vi "TLB Native Dynamic Events ver 0.26bvi.vi"() -> ()   [LabVIEW 2018] (continued)
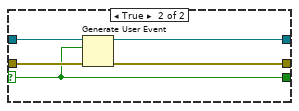
[diagram p2: hidden frame]
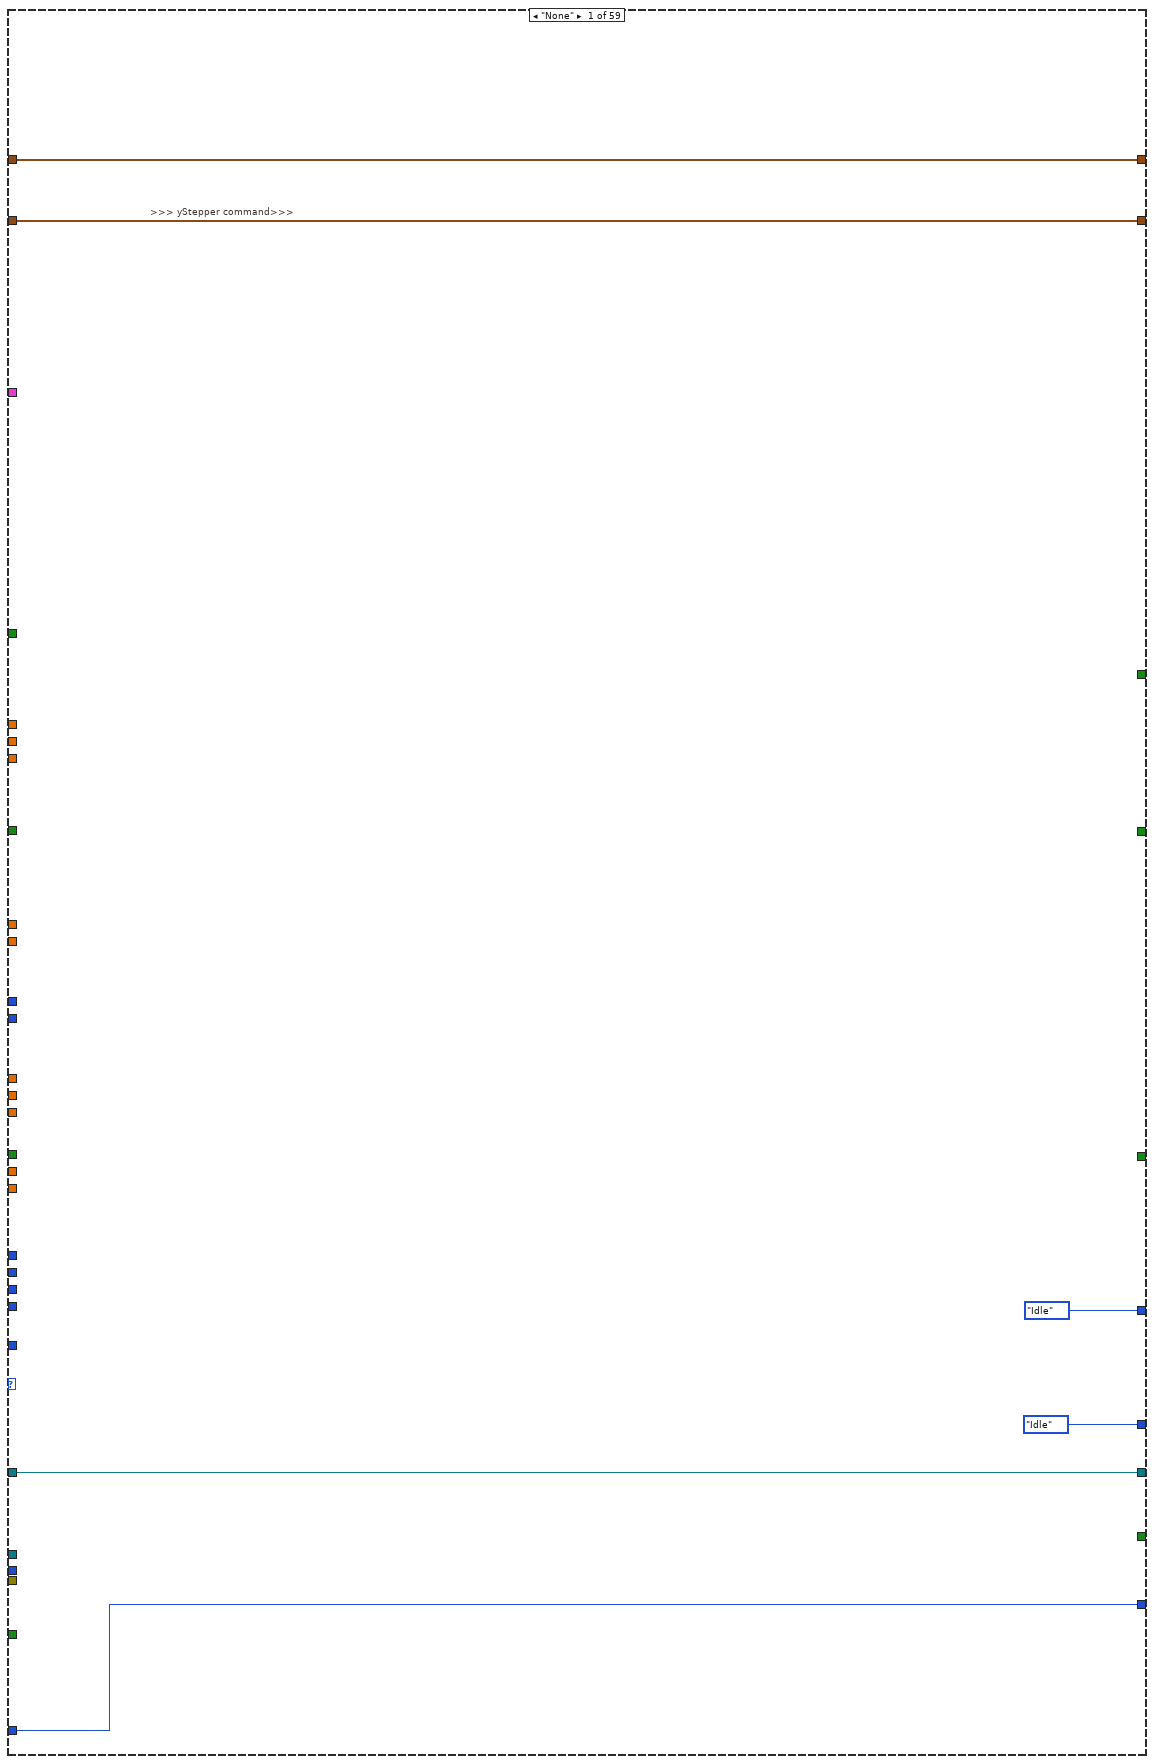
[diagram p5: hidden frame]
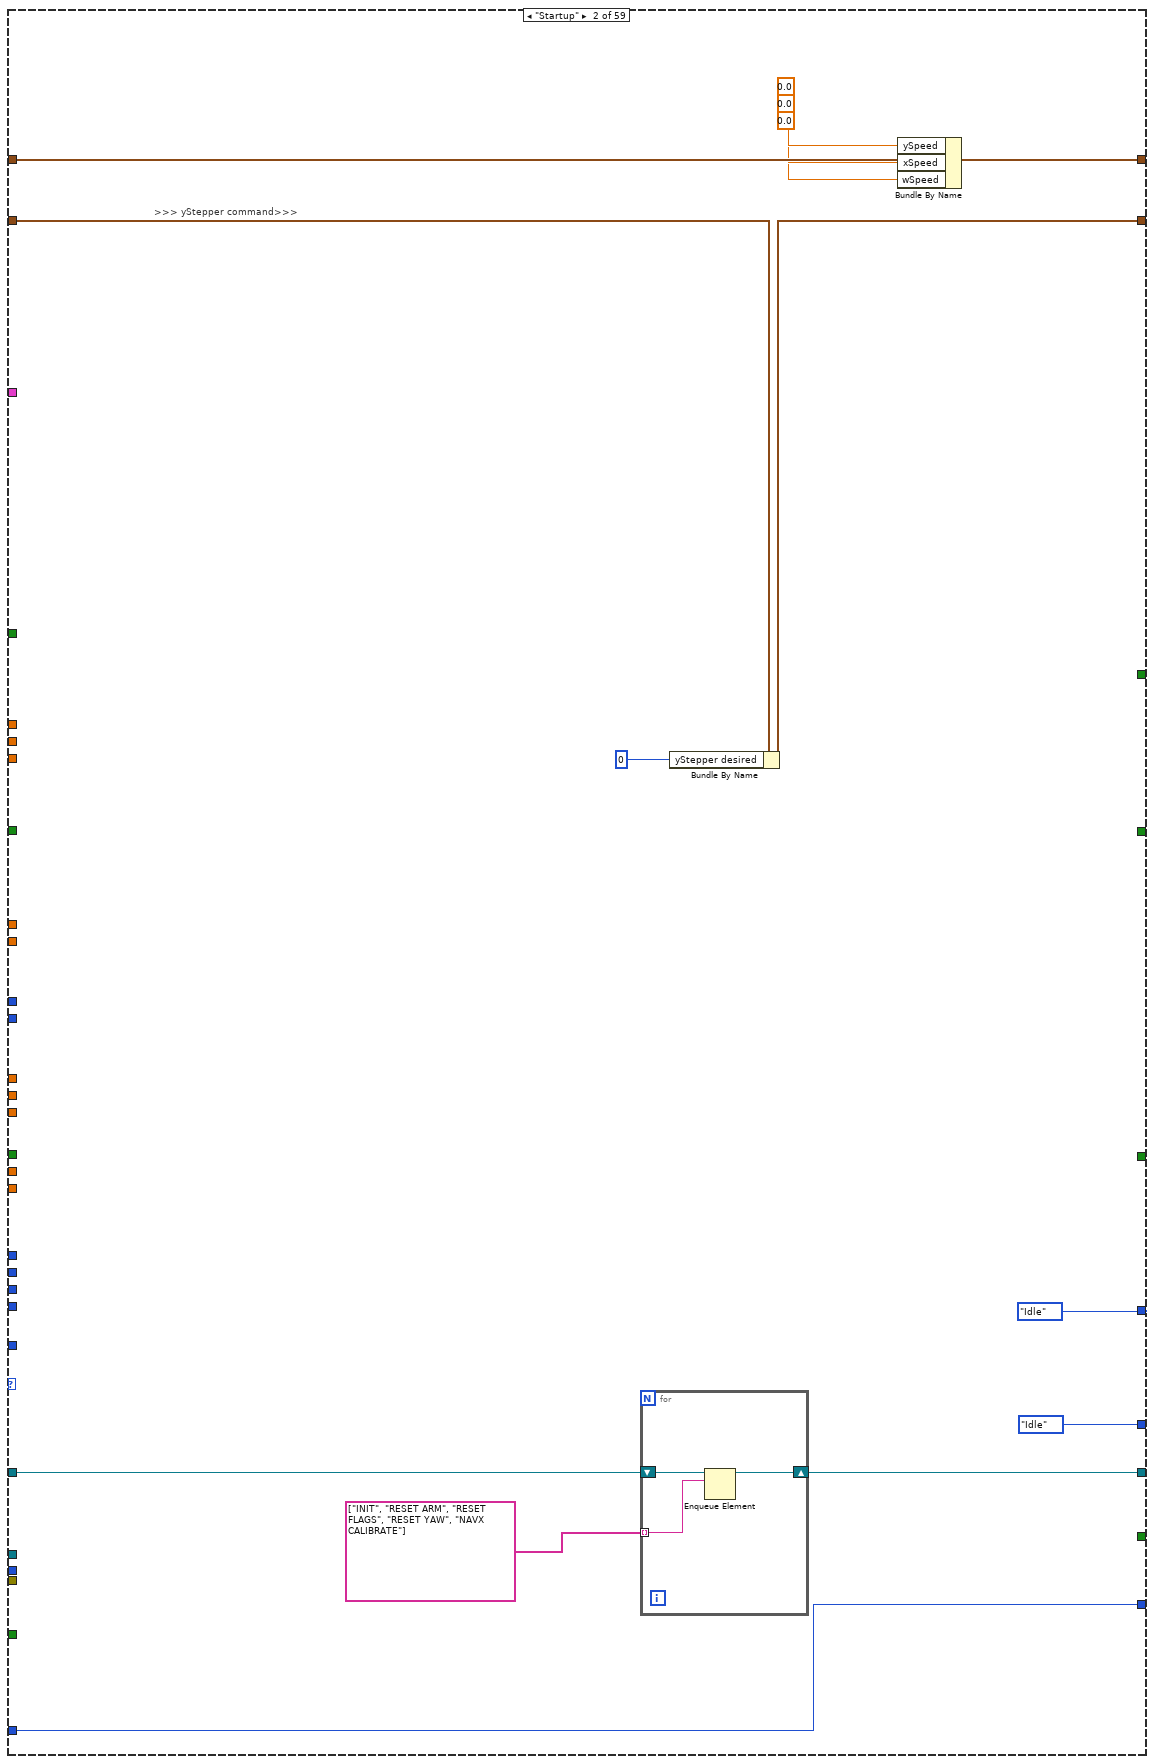
[diagram p6: hidden frame]
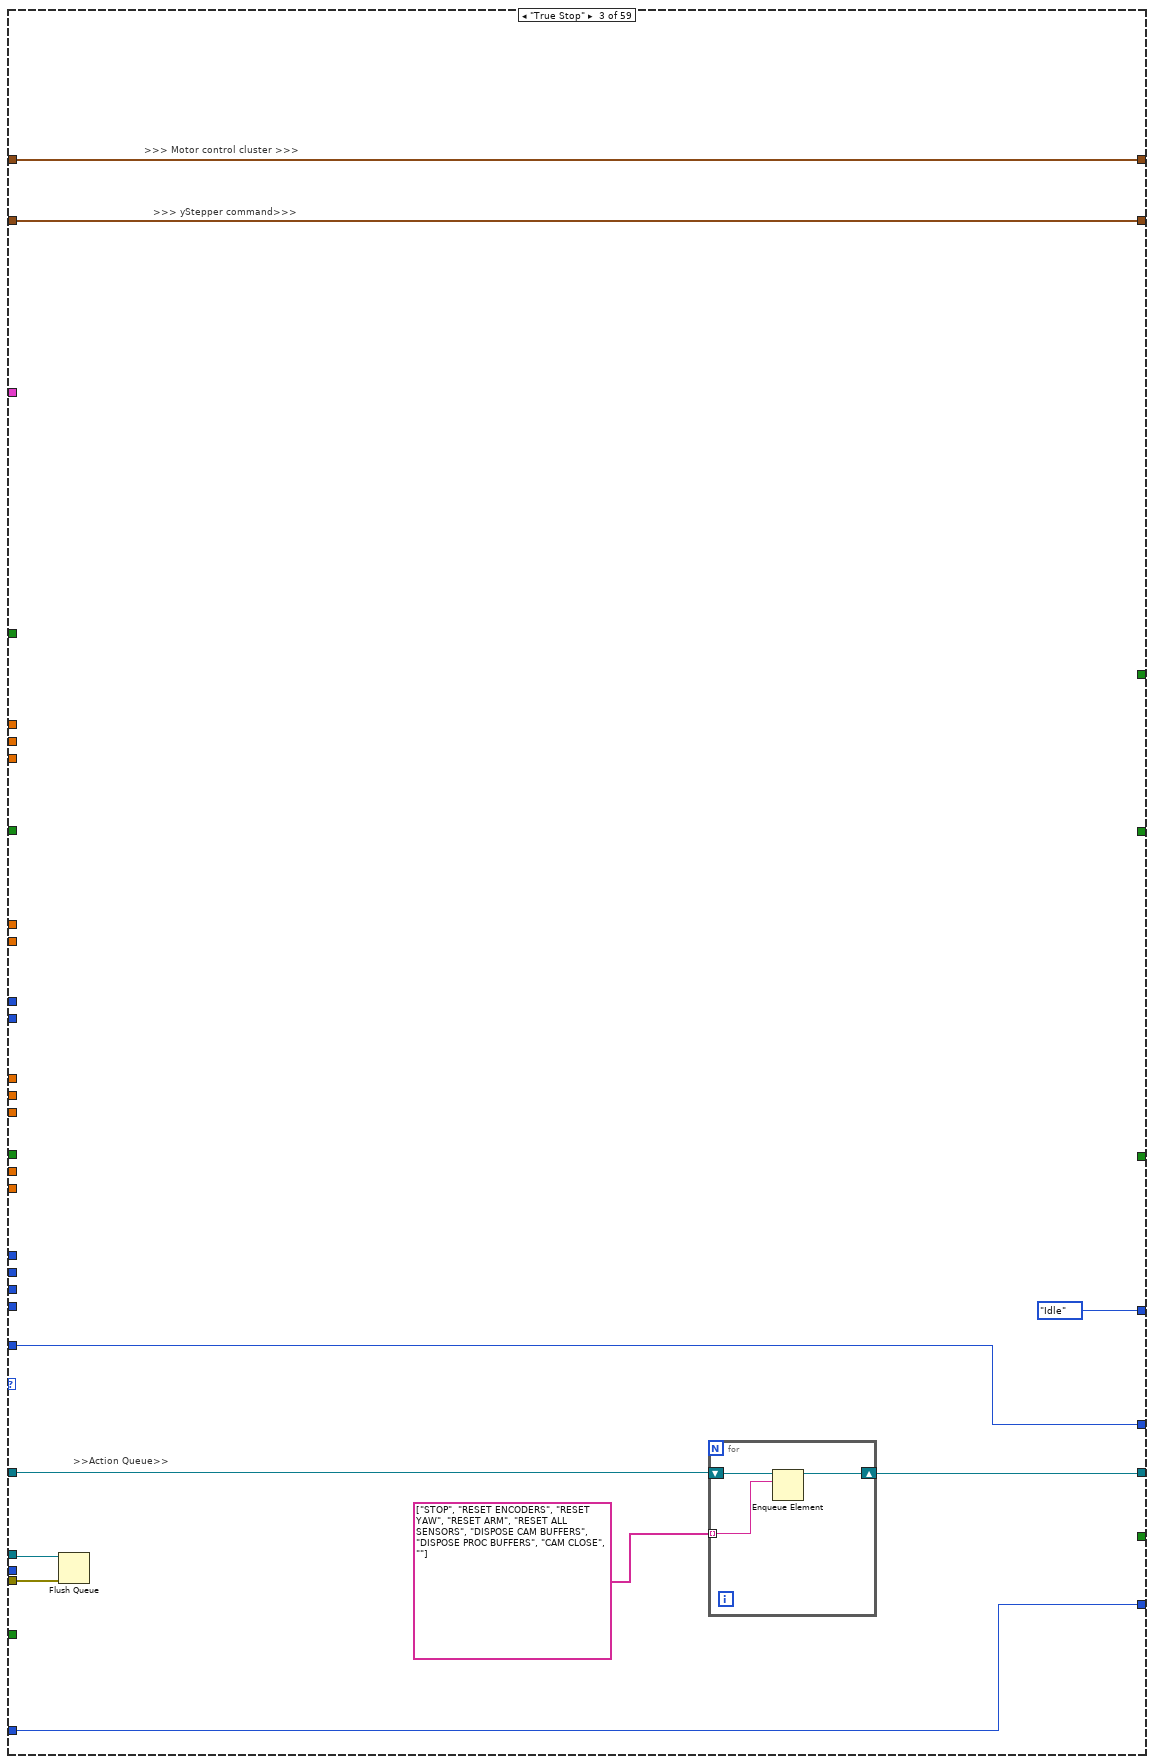
[diagram p7: hidden frame]
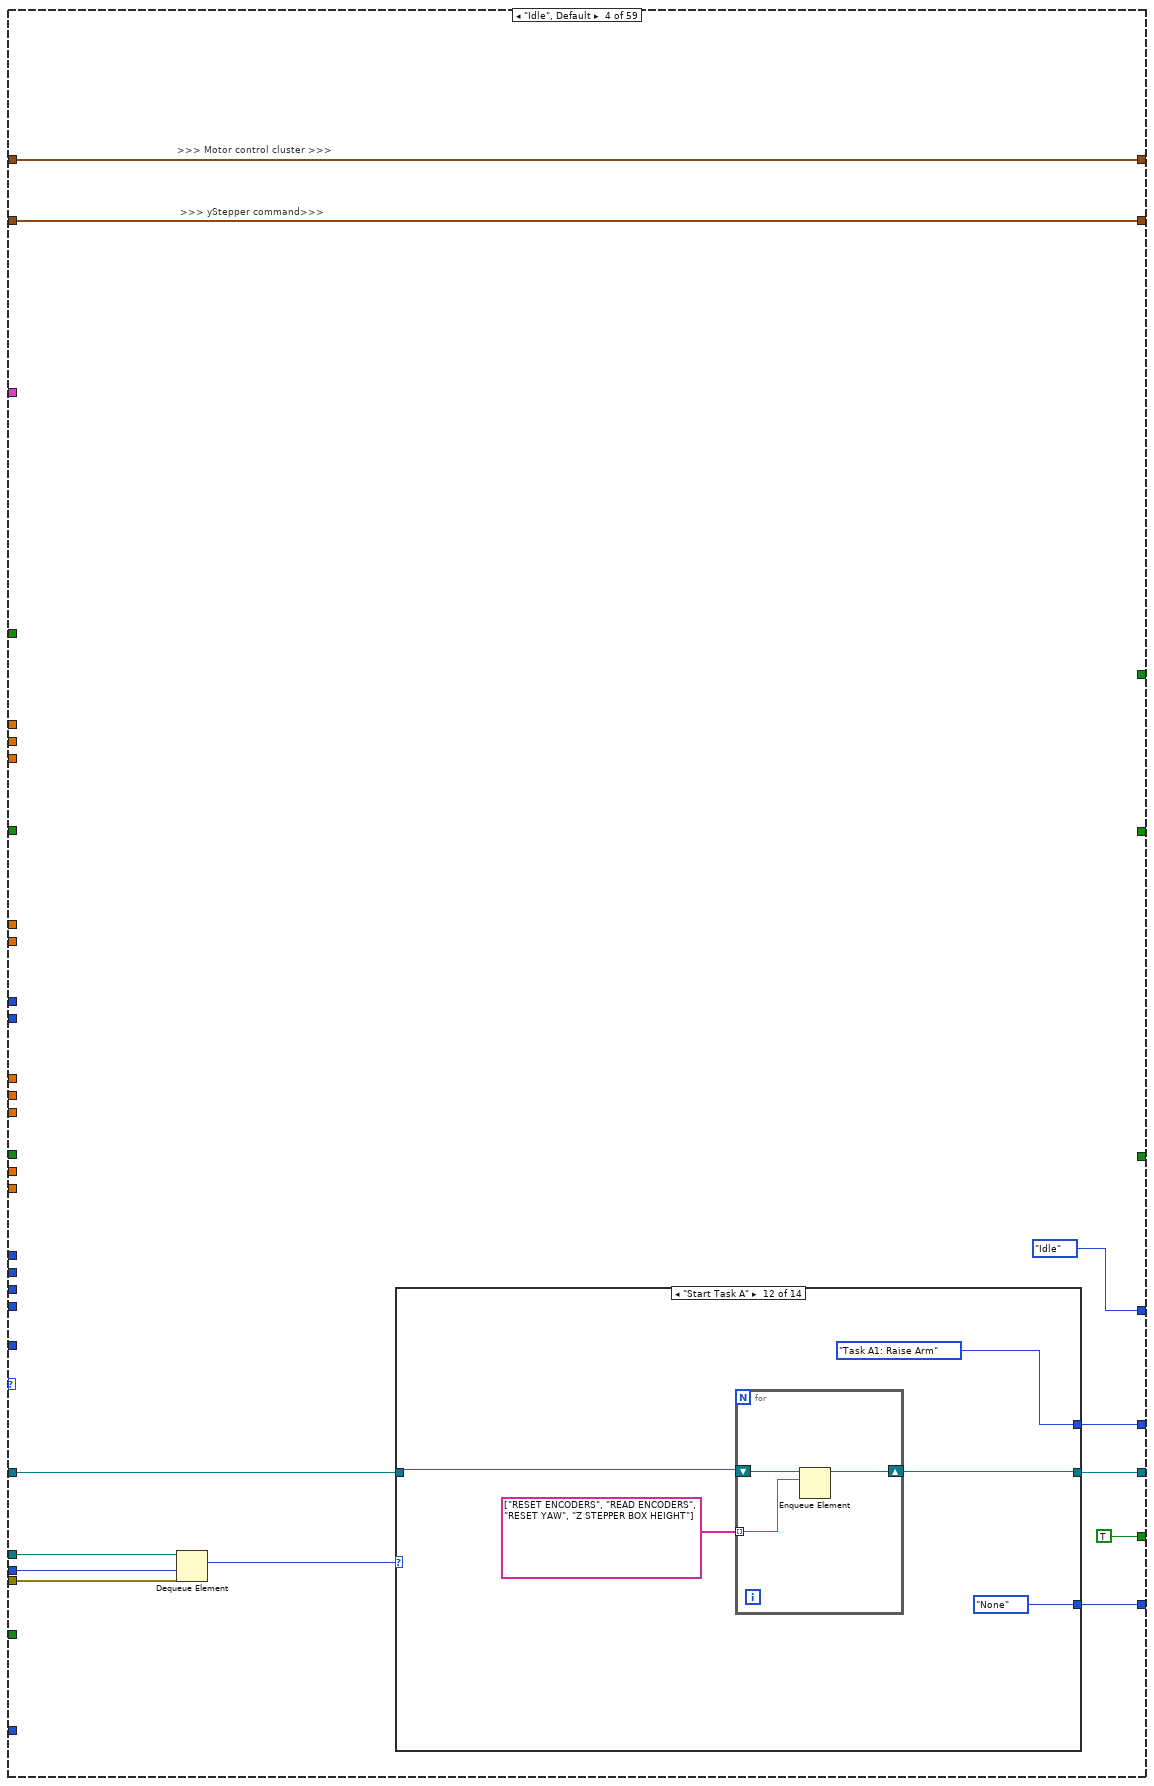
[diagram p8: hidden frame]
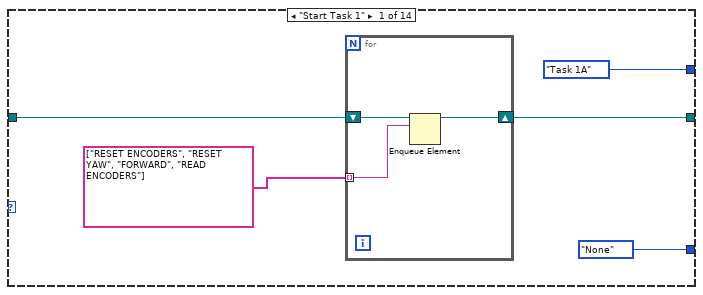
[diagram p9: hidden frame]
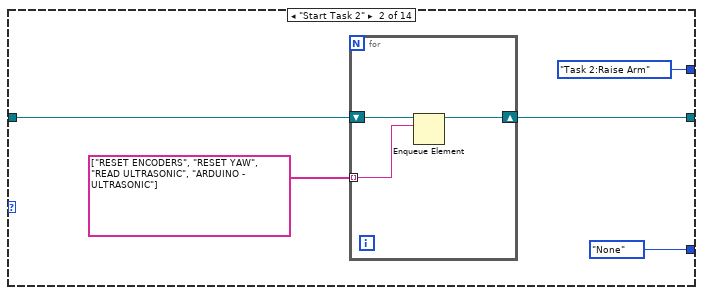
[diagram p10: hidden frame]
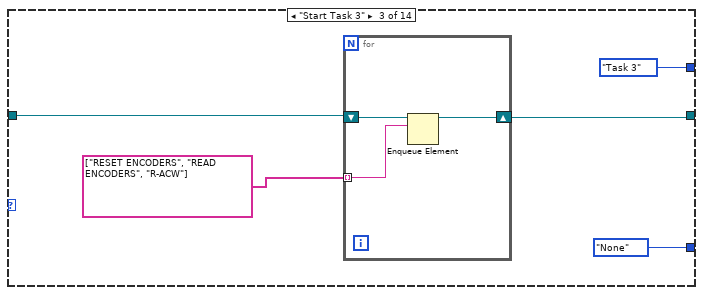
[diagram p11: hidden frame]
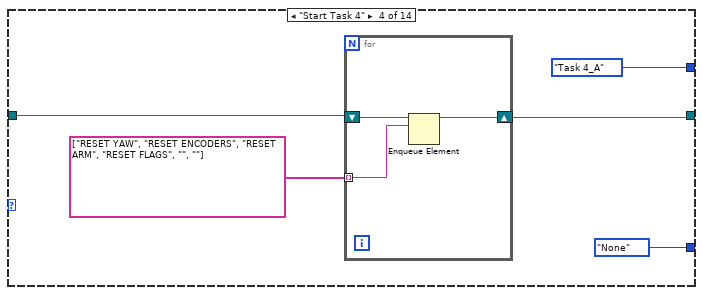
[diagram p12: hidden frame]
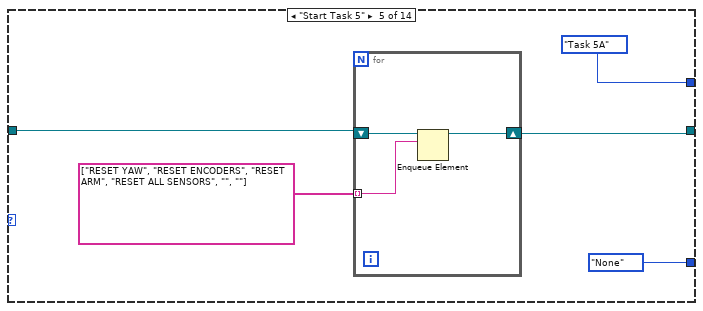
[diagram p13: hidden frame]
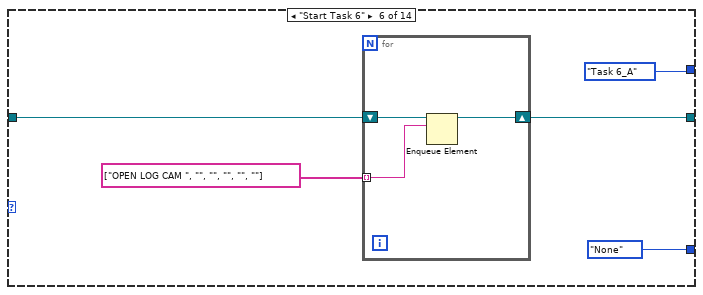
[diagram p14: hidden frame]
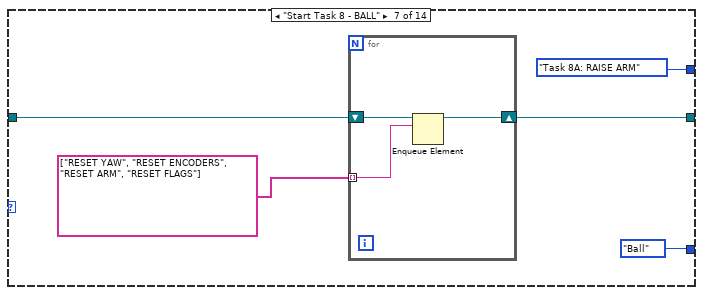
[diagram p15: hidden frame]
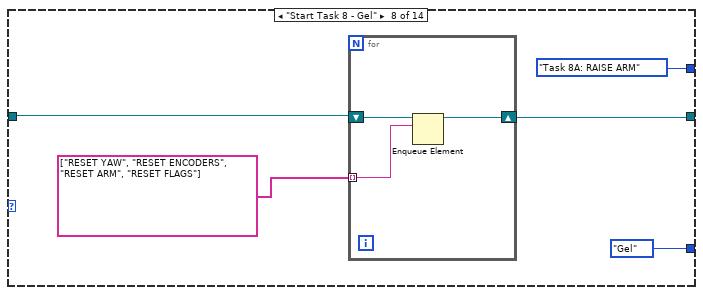
[diagram p16: hidden frame]
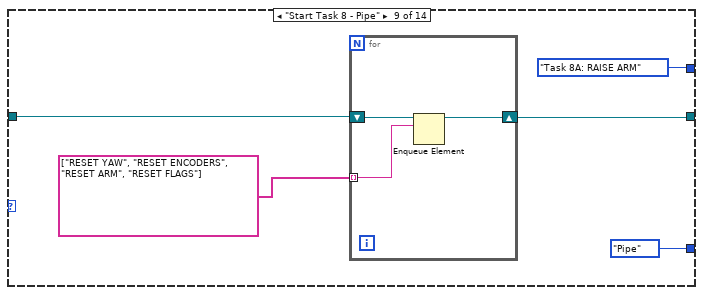
[diagram p17: hidden frame]
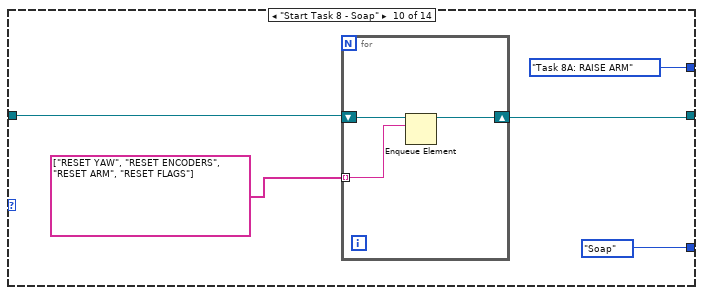
[diagram p18: hidden frame]
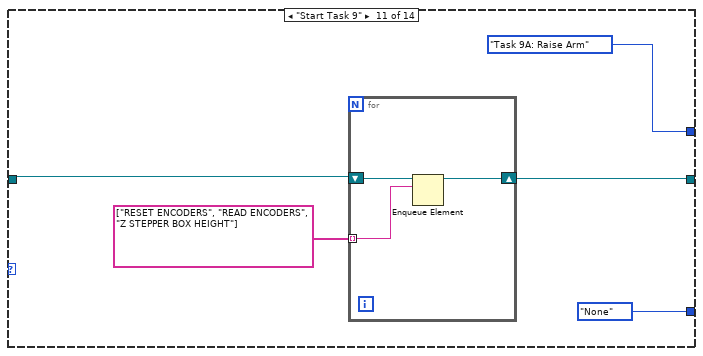
[diagram p19: hidden frame]
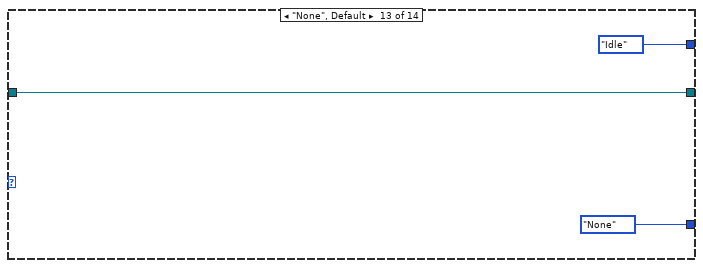
[diagram p20: hidden frame]
              tunnel: w2683 -> [w2693 _]
              frame "Start Task 1", Default {
                # ">> WIill proceed to part ii if not manual override >>"
                # ">>If ENABLE or Trigger is set to true>>"
                n864 = Or(x=w2693, y=w2694) -> (x .or. y?=w2695:bool)
                n865 = case shown="False" w2693 {
                  tunnel: [w2706 w2712] -> w2701
                  tunnel: w2700 -> [w2705 w2711]
                  frame False {
                    n866 = for {
                      shift-right: [w2708] -> w2706
                      shift-left: w2705 -> [w2709]
                      tunnel: string[] ["CAM ACQ", "START TIMER"] ("element") -> [w2707] mode=indexing
                      n867 = Enqueue Element(queue=w2709, element=w2707) -> (queue out=w2708:refnum<queue>)  [unwired: 2 in, 2 out]
                    }
                  }
                  frame True {
                    n868 = for {
                      shift-right: [w2714] -> w2712
                      shift-left: w2711 -> [w2715]
                      tunnel: string[] ["CLOSE CAM", "SET TIMER 5", "", "", "", ""] -> [w2713] mode=indexing
                      n869 = Enqueue Element(queue=w2715, element=w2713) -> (queue out=w2714:refnum<queue>)  [unwired: 2 in, 2 out]
                    }
                  }
                }
                n870 = Select(t=State_Type_Definitions."True Stop" ("Enum"), s=w2694, f=State_Type_Definitions."Task 9R: PROCESS COLOUR" ("Enum")) -> (s? t:f=w2697:T17)
                n871 = Select(t=w2697, s=w2695, f=State_Type_Definitions."Task 9Q: SCAN IMAGE" ("Enum")) -> (s? t:f=w2703:T17)
              }
              frame "Exit" {
                n872 = for {
                  shift-right: [w2722] -> w2719
                  shift-left: w2716 -> [w2723]
                  tunnel: string[] ["STOP", "RESET ENCODERS", "RESET YAW", ""] -> [w2721] mode=indexing
                  n873 = Enqueue Element(queue=w2723, element=w2721) -> (queue out=w2722:refnum<queue>)  [unwired: 2 in, 2 out]
                }
              }
            }
          }
          frame "Task 9R: PROCESS COLOUR" {
            # ">> Item Selection Bias >>"
            # ">>> Motor control cluster >>>"
            # ">>> yStepper command>>>"
            n874 = Dequeue Element(queue=w2729, timeout in ms (-1)=w2730, error in (no error)=w2731) -> (element=w2733:T9)  [unwired: 3 out]
            n875 = case shown="\"Start Task 1\", Default" w2733 {
              tunnel: w2727 -> [w2739 _]
              tunnel: [w2746 State_Type_Definitions."True Stop" ("Enum")] -> w2725
              tunnel: w2732 -> [w2738 _]
              tunnel: w2728 -> [w2745 w2762]
              tunnel: [w2744 w2763] -> w2724
              tunnel: [State_Type_Definitions."Idle" ("Enum") State_Type_Definitions."Shutdown" ("Enum")] -> w2726
              frame "Start Task 1", Default {
                n876 = case shown="False" w2739 {
                  tunnel: w2745 -> [w2749 w2756]
                  tunnel: [w2750 w2755] -> w2744
                  frame False {
                    n877 = for {
                      tunnel: string[] ["START TIMER", "COLOUR PROCESSING", ""] ("element") -> [w2751] mode=indexing
                      shift-right: [w2753] -> w2750
                      shift-left: w2749 -> [w2752]
                      n878 = Enqueue Element(queue=w2752, element=w2751) -> (queue out=w2753:refnum<queue>)  [unwired: 2 in, 2 out]
                    }
                  }
                  frame True {
                    n879 = for {
                      shift-right: [w2758] -> w2755
                      shift-left: w2756 -> [w2759]
                      tunnel: string[] ["CLOSE CAM", "DISPOSE BUFFERS", "RESET ENCODERS", "RESET YAW", "RESET FLAGS", ""] -> [w2757] mode=indexing
                      n880 = Enqueue Element(queue=w2759, element=w2757) -> (queue out=w2758:refnum<queue>)  [unwired: 2 in, 2 out]
                    }
                  }
                }
                n881 = Or(x=w2739, y=w2738) -> (x .or. y?=w2737:bool)
                n882 = Select(t=State_Type_Definitions."True Stop" ("Enum"), s=w2738, f=State_Type_Definitions."True Stop" ("Enum")) -> (s? t:f=w2740:T17)
                n883 = Select(t=w2740, s=w2737, f=State_Type_Definitions."Task 9R: PROCESS COLOUR" ("Enum")) -> (s? t:f=w2746:T17)
              }
              frame "Exit" {
                n884 = for {
                  shift-right: [w2766] -> w2763
                  shift-left: w2762 -> [w2767]
                  tunnel: string[] ["STOP", "RESET ENCODERS", "RESET YAW", "ARDUINO MODE 0"] -> [w2765] mode=indexing
                  n885 = Enqueue Element(queue=w2767, element=w2765) -> (queue out=w2766:refnum<queue>)  [unwired: 2 in, 2 out]
                }
              }
            }
          }
          frame "Task A1: Raise Arm" {
            # ">>> Motor control cluster >>>"
            # ">> Stepper height reeached >>"
            # ">>> yStepper command>>>"
            # ">> Manual override >>"
            n886 = Dequeue Element(queue=w2779, timeout in ms (-1)=w2774, error in (no error)=w2778) -> (element=w2782:T9)  [unwired: 3 out]
            n887 = Equal?(x=w2776, y=u8 50) -> (x = y?=w2780:bool)
            n888 = case shown="\"Start Task 1\", Default" w2782 {
              tunnel: [w2793 State_Type_Definitions."True Stop" ("Enum")] -> w2772
              tunnel: [w2791 w2808] -> w2771
              tunnel: w2775 -> [w2790 _]
              tunnel: w2777 -> [w2784 _]
              tunnel: [State_Type_Definitions."Idle" ("Enum") State_Type_Definitions."Shutdown" ("Enum")] -> w2773
              tunnel: w2780 -> [w2783 _]
              frame "Start Task 1", Default {
                # ">> WIill proceed to part ii if not manual override >>"
                # ">>If ENABLE or Trigger is set to true>>"
                n889 = Or(x=w2783, y=w2784) -> (x .or. y?=w2785:bool)
                n890 = case shown="False" w2783 {
                  tunnel: [w2796 w2802] -> w2791
                  tunnel: w2790 -> [w2795 w2801]
                  frame False {
                    n891 = for {
                      shift-right: [w2798] -> w2796
                      shift-left: w2795 -> [w2799]
                      tunnel: string[] ["Z STEPPER BOX HEIGHT", "READ STEPPER VALUES"] ("element") -> [w2797] mode=indexing
                      n892 = Enqueue Element(queue=w2799, element=w2797) -> (queue out=w2798:refnum<queue>)  [unwired: 2 in, 2 out]
                    }
                  }
                  frame True {
                    n893 = for {
                      shift-right: [w2804] -> w2802
                      shift-left: w2801 -> [w2805]
                      tunnel: string[] ["ARDUINO - ULTRASONIC", "READ NAVX", "RESET FLAGS", "", "", ""] -> [w2803] mode=indexing
                      n894 = Enqueue Element(queue=w2805, element=w2803) -> (queue out=w2804:refnum<queue>)  [unwired: 2 in, 2 out]
                    }
                  }
                }
                n895 = Select(t=State_Type_Definitions."True Stop" ("Enum"), s=w2784, f=State_Type_Definitions."Task A2: Rotate to Angle" ("Enum")) -> (s? t:f=w2787:T17)
                n896 = Select(t=w2787, s=w2785, f=State_Type_Definitions."Task A1: Raise Arm" ("Enum")) -> (s? t:f=w2793:T17)
              }
              frame "Exit" {
                n897 = for {
                  shift-right: [w2811] -> w2808
                  shift-left: _ -> [w2812]
                  tunnel: string[] ["STOP", "RESET ENCODERS", "RESET YAW", ""] -> [w2810] mode=indexing
                  n898 = Enqueue Element(queue=w2812, element=w2810) -> (queue out=w2811:refnum<queue>)  [unwired: 2 in, 2 out]
                }
              }
            }
          }
          frame "Task A2: Rotate to Angle" {
            # ">>> Motor control cluster >>>"
            # ">>> yStepper command>>>"
            n899 = Dequeue Element(queue=w2826, timeout in ms (-1)=w2825, error in (no error)=w2824) -> (element=w2828:T9)  [unwired: 3 out]
            n900 = In Range and Coerce(upper limit=65.0, x=w2818, lower limit=58.0) -> (In Range?=w2815:bool)  [unwired: 1 out]
            n901 = case shown="\"Start Task 1\", Default" w2828 {
              tunnel: w2819 -> [w2831 _]
              tunnel: [w2839 State_Type_Definitions."True Stop" ("Enum")] -> w2821
              tunnel: w2827 -> [w2837 w2855]
              tunnel: [w2836 w2854] -> w2820
              tunnel: [State_Type_Definitions."Idle" ("Enum") State_Type_Definitions."Shutdown" ("Enum")] -> w2822
              tunnel: w2815 -> [w2829 _]
              frame "Start Task 1", Default {
                n902 = Or(x=w2829, y=w2831) -> (x .or. y?=w2830:bool)
                n903 = case shown="True" w2829 {
                  tunnel: w2837 -> [w2842 w2848]
                  tunnel: [w2841 w2846] -> w2836
                  frame False {
                    n904 = for {
                      shift-right: [w2844] -> w2841
                      shift-left: w2842 -> [w2845]
                      tunnel: string[] ["READ NAVX", "R-CW", "READ ULTRASONIC"] ("element") -> [w2843] mode=indexing
                      n905 = Enqueue Element(queue=w2845, element=w2843) -> (queue out=w2844:refnum<queue>)  [unwired: 2 in, 2 out]
                    }
                  }
                  frame True {
                    n906 = for {
                      shift-right: [w2850] -> w2846
                      shift-left: w2848 -> [w2851]
                      tunnel: string[] ["STOP", "RESET ENCODERS", "RESET YAW", "READ IR", "ARDUINO - ULTRASONIC"] -> [w2849] mode=indexing
                      n907 = Enqueue Element(queue=w2851, element=w2849) -> (queue out=w2850:refnum<queue>)  [unwired: 2 in, 2 out]
                    }
                  }
                }
                n908 = Select(t=State_Type_Definitions."True Stop" ("Enum"), s=w2831, f=State_Type_Definitions."Task A3: Move Forward") -> (s? t:f=w2833:T17)
                n909 = Select(t=w2833, s=w2830, f=State_Type_Definitions."Task A2: Rotate to Angle" ("Enum")) -> (s? t:f=w2839:T17)
              }
              frame "Exit" {
                n910 = for {
                  shift-right: [w2858] -> w2854
                  shift-left: w2855 -> [w2859]
                  tunnel: string[] ["STOP", "RESET ENCODERS", "RESET YAW", ""] -> [w2857] mode=indexing
                  n911 = Enqueue Element(queue=w2859, element=w2857) -> (queue out=w2858:refnum<queue>)  [unwired: 2 in, 2 out]
                }
              }
            }
          }
          frame "Task A3: Move Forward" {
            (unwired) 50.0 ("y")
            (unwired) 15.0 ("y")
            # ">> Item Selection Bias >>"
            # ">> Wall detected >>"
            # ">> Manual override >>"
            # ">>> Motor control cluster >>>"
            # ">>Table or wall detectected>>"
            # ">>Action Queue>>"
            # ">>> yStepper command>>>"
            n912 = Dequeue Element(queue=w2875, timeout in ms (-1)=w2874, error in (no error)=w2873) -> (element=w2876:T9)  [unwired: 3 out]
            n913 = Less?(x=w2862, y=100.0) -> (x < y?=w2863:bool)
            n914 = Not Equal To 0?(x=w2862) -> (x != 0?=w2861:bool)
            n915 = And(x=w2861, y=w2863) -> (x .and. y?=w2860:bool)
            n916 = case shown="\"Start Task 1\", Default" w2876 {
              tunnel: w2871 -> [w2877 _]
              tunnel: [w2887 State_Type_Definitions."True Stop" ("Enum")] -> w2868
              tunnel: w2872 -> [w2885 w2903]
              tunnel: [w2884 w2902] -> w2867
              tunnel: [State_Type_Definitions."Idle" ("Enum") State_Type_Definitions."Shutdown" ("Enum")] -> w2870
              tunnel: w2860 -> [w2878 _]
              frame "Start Task 1", Default {
                n917 = Or(x=w2877, y=w2878) -> (x .or. y?=w2879:bool)
                n918 = case shown="False" w2878 {
                  tunnel: w2885 -> [w2890 w2896]
                  tunnel: [w2889 w2894] -> w2884
                  frame False {
                    n919 = for {
                      shift-right: [w2892] -> w2889
                      shift-left: w2890 -> [w2893]
                      tunnel: string[] ["READ IR", "FORWARD - IR ASSIST", "READ ULTRASONIC"] ("element") -> [w2891] mode=indexing
                      n920 = Enqueue Element(queue=w2893, element=w2891) -> (queue out=w2892:refnum<queue>)  [unwired: 2 in, 2 out]
                    }
                  }
                  frame True {
                    n921 = for {
                      shift-right: [w2898] -> w2894
                      shift-left: w2896 -> [w2899]
                      tunnel: string[] ["STOP", "RESET ENCODERS", "RESET YAW", ""] -> [w2897] mode=indexing
                      n922 = Enqueue Element(queue=w2899, element=w2897) -> (queue out=w2898:refnum<queue>)  [unwired: 2 in, 2 out]
                    }
                  }
                }
                n923 = Select(t=State_Type_Definitions."True Stop" ("Enum"), s=w2877, f=State_Type_Definitions."Task A4: Rotate CW 90") -> (s? t:f=w2881:T17)
                n924 = Select(t=w2881, s=w2879, f=State_Type_Definitions."Task A3: Move Forward" ("Enum")) -> (s? t:f=w2887:T17)
              }
              frame "Exit" {
                n925 = for {
                  shift-right: [w2906] -> w2902
                  shift-left: w2903 -> [w2907]
                  tunnel: string[] ["STOP", "RESET ENCODERS", "RESET YAW", ""] -> [w2905] mode=indexing
                  n926 = Enqueue Element(queue=w2907, element=w2905) -> (queue out=w2906:refnum<queue>)  [unwired: 2 in, 2 out]
                }
              }
            }
          }
          frame "Task A4: Rotate CW 90" {
            # ">>> Motor control cluster >>>"
            # ">>> yStepper command>>>"
            # ">> Item Selection Bias >>"
            n927 = Less?(x=w2911, y=-40.0) -> (x < y?=w2909:bool)
            n928 = Dequeue Element(queue=w2917, timeout in ms (-1)=w2916, error in (no error)=w2915) -> (element=w2919:T9)  [unwired: 3 out]
            n929 = case shown="\"Start Task 1\", Default" w2919 {
              tunnel: w2909 -> [w2925 _]
              tunnel: [w2932 State_Type_Definitions."True Stop" ("Enum")] -> w2913
              tunnel: w2914 -> [w2924 _]
              tunnel: w2918 -> [w2931 w2948]
              tunnel: [w2930 w2949] -> w2908
              tunnel: [State_Type_Definitions."Idle" ("Enum") State_Type_Definitions."Shutdown" ("Enum")] -> w2912
              frame "Start Task 1", Default {
                n930 = case shown="True" w2925 {
                  tunnel: w2931 -> [w2935 w2942]
                  tunnel: [w2936 w2941] -> w2930
                  frame False {
                    n931 = for {
                      tunnel: string[] ["READ ENCODERS", "R-CW"] ("element") -> [w2937] mode=indexing
                      shift-right: [w2939] -> w2936
                      shift-left: w2935 -> [w2938]
                      n932 = Enqueue Element(queue=w2938, element=w2937) -> (queue out=w2939:refnum<queue>)  [unwired: 2 in, 2 out]
                    }
                  }
                  frame True {
                    n933 = for {
                      shift-right: [w2944] -> w2941
                      shift-left: w2942 -> [w2945]
                      tunnel: string[] ["STOP", "RESET ENCODERS", "RESET FLAGS", "RESET YAW", "READ IR", ""] -> [w2943] mode=indexing
                      n934 = Enqueue Element(queue=w2945, element=w2943) -> (queue out=w2944:refnum<queue>)  [unwired: 2 in, 2 out]
                    }
                  }
                }
                n935 = Or(x=w2925, y=w2924) -> (x .or. y?=w2923:bool)
                n936 = Select(t=State_Type_Definitions."True Stop" ("Enum"), s=w2924, f=State_Type_Definitions."Task A3: Move Forward" ("Enum")) -> (s? t:f=w2926:T17)
                n937 = Select(t=w2926, s=w2923, f=State_Type_Definitions."Task A4: Rotate CW 90" ("Enum")) -> (s? t:f=w2932:T17)
              }
              frame "Exit" {
                n938 = for {
                  shift-right: [w2952] -> w2949
                  shift-left: w2948 -> [w2953]
                  tunnel: string[] ["STOP", "RESET ENCODERS", "RESET YAW", "ARDUINO MODE 0"] -> [w2951] mode=indexing
                  n939 = Enqueue Element(queue=w2953, element=w2951) -> (queue out=w2952:refnum<queue>)  [unwired: 2 in, 2 out]
                }
              }
            }
          }
        }
        "Object Detection" <- w313
        "Ultrasonic sensors" <- w336
        "Encoder values" <- w325
        "Stepper position values" <- w309
        "NAVX Values" <- w307
        "IR Sensors" <- w299
        "Line sensors" <- w294
        "Time cluster" <- w305
        "Box Colour Detection" <- w287
      }
    }
    "Object recognition mode" <- w220
    "Front Ultrasonic obstruct" <- w217
    "Front IR obstruct" <- w216
    "Table IR obstruct" <- w215
    n940 = local write "Green LED"(w230) -> ()
  }
  n941 = while {
    stop <- w3794 stop-if-true
    n942 = call "MOTOR CONTROL WITH PID AE.vi"("AE Mode"=MOTOR_CONTROL_WITH_PID_AE_DATA_MODE_TYPE_DEF."Read from AE") -> ("Speed & distance"=→"Speed & distance":T14)  [unwired: 3 in]
    n943 = call "FGV Bool.vi"("Init/Read/Write State"=States_for_Action_Engine."Read") -> ("Output node"=w3794:bool)  [unwired: 2 in, 1 out]
    n944 = Wait (ms)(milliseconds to wait=u32 5) -> ()  [unwired: 1 out]
  }
  n945 = call <vilib>:"DIO Close.vi"("error in (no error)"=w23, "DIO Info In"=w26) -> ()  [unwired: 9 in, 1 out]
  n946 = call <vilib>:"DIO Close.vi"("error in (no error)"=w33, "DIO Info In"=w35) -> ()  [unwired: 9 in, 1 out]
  n947 = call <vilib>:"NavX Close.vi"("error in (no error)"=w10, "NavX Info In"=w9) -> ()  [unwired: 9 in, 1 out]
  n948 = call <vilib>:"DIO Close.vi"("error in (no error)"=w28, "DIO Info In"=w30) -> ()  [unwired: 9 in, 1 out]
  n949 = call <vilib>:"DIO Close.vi"("error in (no error)"=w17, "DIO Info In"=w18) -> ()  [unwired: 9 in, 1 out]
  n950 = call <vilib>:"DIO Close.vi"("error in (no error)"=w12, "DIO Info In"=w13) -> ()  [unwired: 9 in, 1 out]
  n951 = Merge Errors "Merge Errors"(w63, w62) -> (w45:errorcluster)
  n952 = Merge Errors(w49, w45) -> (w44:errorcluster)
  n953 = Destroy User Event(user event=w67, error in=w44) -> ()  [unwired: 1 out]
  n954 = Release Queue(queue=w40, error in (no error)=w44) -> (error out=→"Queue Errors":errorcluster)  [unwired: 1 in, 2 out]
  n955 = Release Queue(queue=w57, error in (no error)=w44) -> ()  [unwired: 1 in, 3 out]
  n956 = Destroy User Event(user event=w66, error in=w44) -> ()  [unwired: 1 out]
  n957 = Unregister For Events(event registration refnum=w58, error in=w44) -> ()  [unwired: 1 out]
